vi "画箭头 - right.vi"(0 "Image 2":T1(plugin-control)=refnum, 5 "距离":dbl, 7 "Rectangle":T3={"Left"=793, "Top"=1130, "Right"=0, "Bottom"=0, "Rotation"=45.0} {"Rotation" format="%.2f"; "Left" scale=0.0..1024.0; "Right" scale=0.0..1024.0}, 9 "abgek":dbl, 11 "error in (no error)":errorcluster caption="错误输入（无错误）", 12 "long":sgl=300.0, 13 "Color 2":u32(colorbox)=16711680) -> (4 "Image out":T1(plugin-control), 15 "error out":errorcluster)   [LabVIEW 2017]
uses:
  <vilib>/Analysis/coordinate.llb/2D Cartesian Coordinate Shift (Array).vi
  <vilib>/Analysis/coordinate.llb/2D Cartesian Coordinate Rotation (Array).vi
  <vilib>/Analysis/NI_AALPro.lvlib
panel:
  in  "Width":u32=23
  out "添加的数组":T2[](array[typedef]) {"Y" format="%.2f"; "X" format="%.2f"}
  in  "Color":u32(colorbox)=16711680
  out "MiddleEndPoint":T2={"X"=892.0, "Y"=1299.75} {"Y" format="%.2f"; "X" format="%.2f"}
  out "MiddleStartPoint":T2={"X"=892.0, "Y"=1159.25} {"Y" format="%.2f"; "X" format="%.2f"}
  out "EndPoint":T2={"X"=892.0, "Y"=1370.0} {"Y" format="%.2f"; "X" format="%.2f"}
  out "StartPoint":T2={"X"=892.0, "Y"=1089.0} {"Y" format="%.2f"; "X" format="%.2f"}
  in  "sss":i32=30
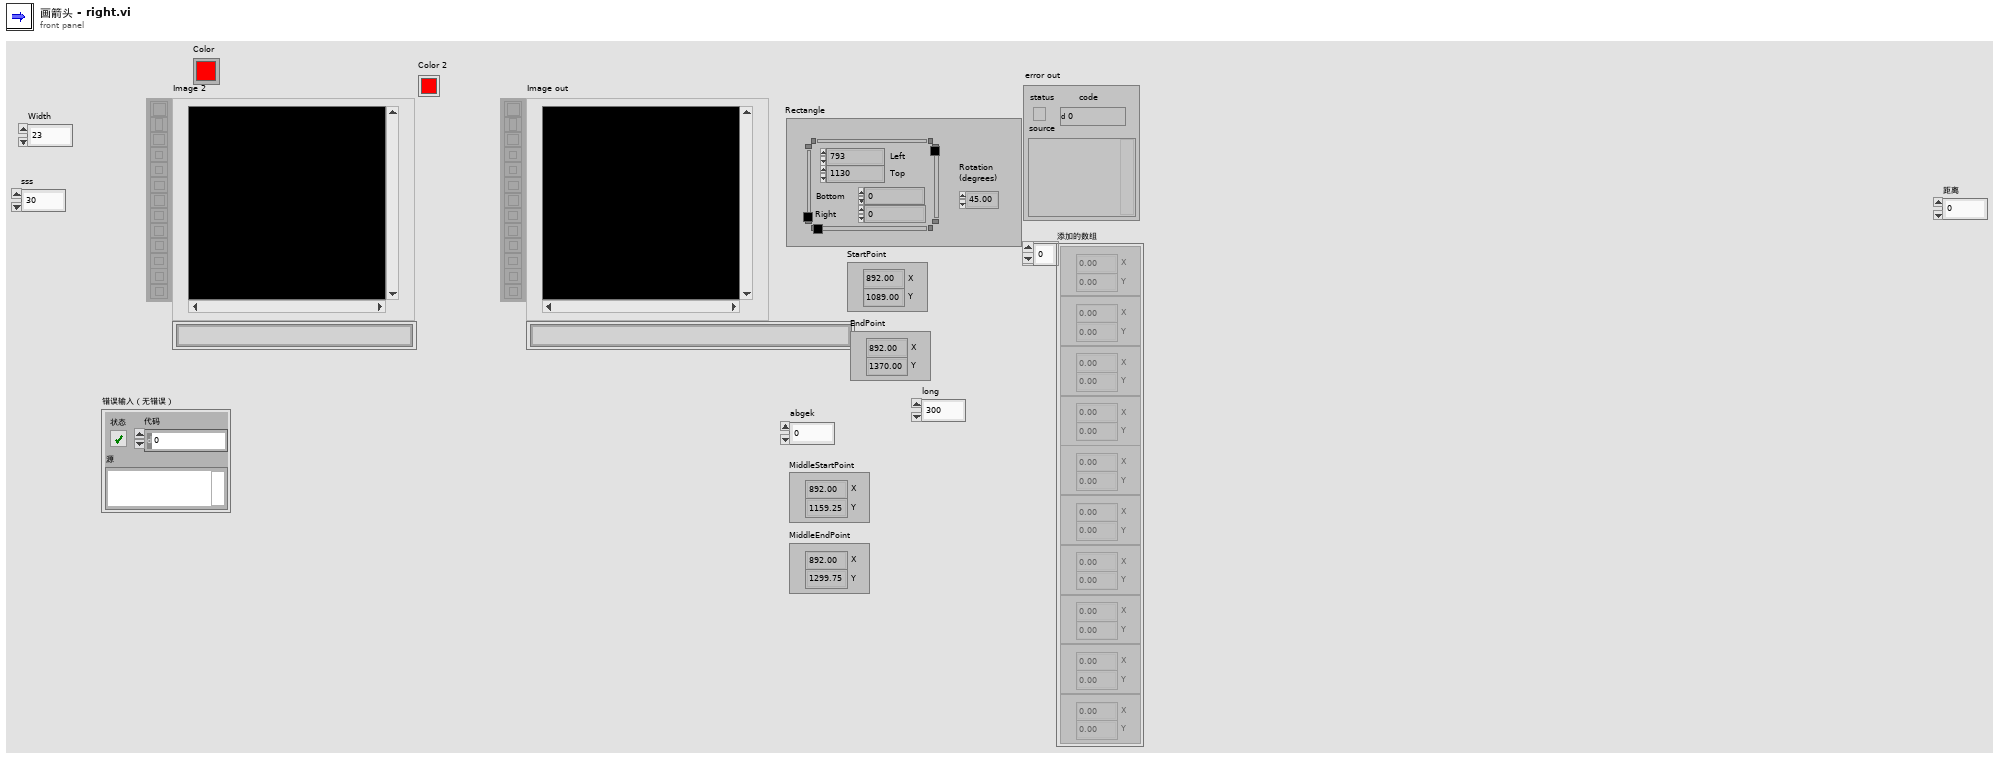
[diagram p1: front panel]
types:
  T1 = typedef "IMAQ Image.ctl" = refnum<image>
  T2 = typedef "IMAQ Point" = cluster{"X":sgl, "Y":sgl}
  T3 = typedef "IMAQ Rectangle" = cluster{"Left":i32, "Top":i32, "Right":i32, "Bottom":i32, "Rotation":dbl}
  T4 = cluster{"Desired Font (Application)":enum16{"User-specified Font", "Application Font", "System Font", "Dialog Font"}, "[User-specified Font]":cluster{"Font Name":string, "Size":i16, "Strikeout?":bool, "Italic?":bool, "Underline?":bool, "Outline?":bool, "Shadow?":bool, "Bold?":bool, "Rotation Angle":dbl}, "Horizontal Alignment":i16, "Vertical Alignment":i16}
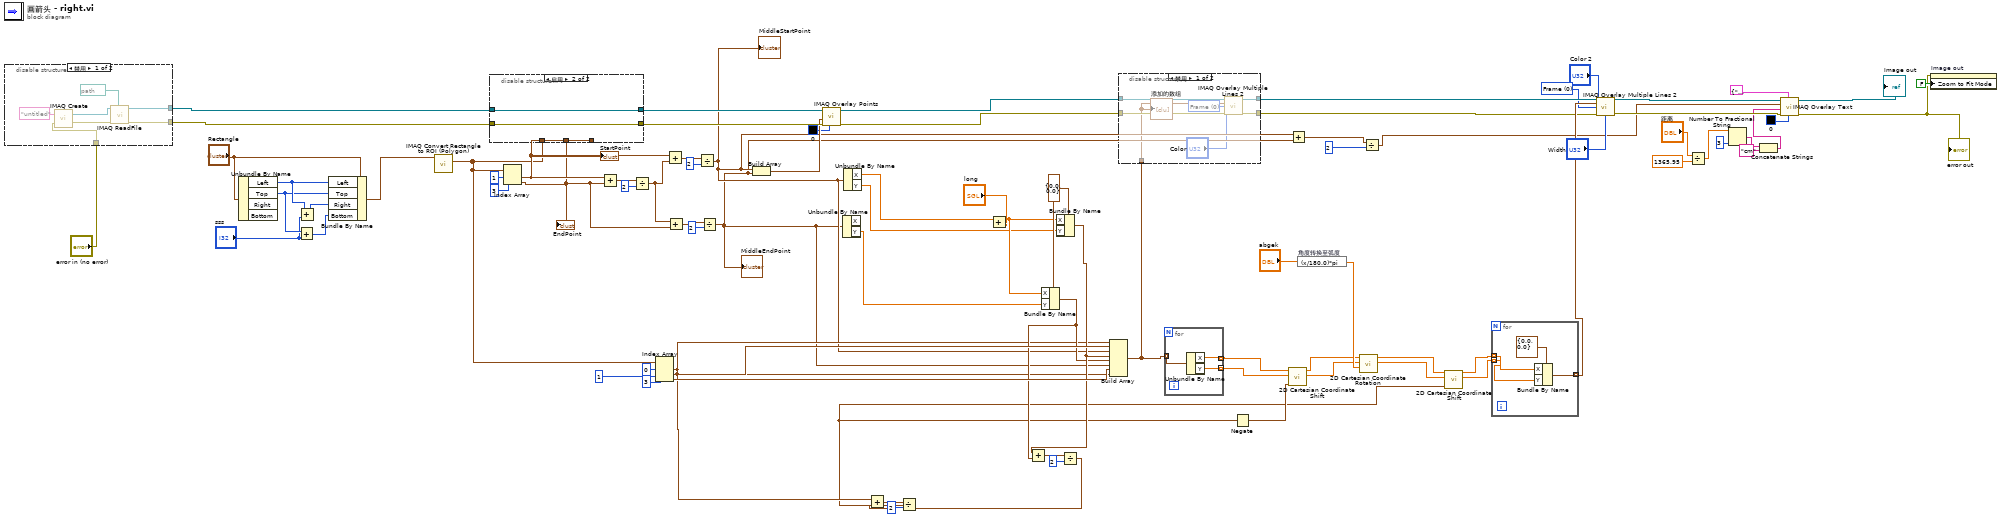
[diagram p0: block diagram]
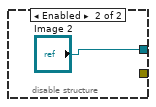
[diagram p2: hidden frame]
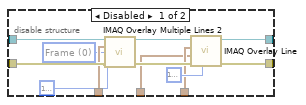
[diagram p4: hidden frame]
diagram:
  w34 = u32 0 items=["Frame", "Fill"] ("Drawing Mode (Frame)")
  w55 = T2 {"X"=0.0, "Y"=0.0} ("元素")
  n1 = disable-structure shown="禁用" {
    disable-tunnel: [w88 "Image 2"] -> w21
    disable-tunnel: [w87 _] -> w20
    disable-tunnel: "error in (no error)" -> [w86 _]
    frame Disabled {
      n2 = call "IMAQ Create"("Image Name"="untitled", "error in (no error)"=w86) -> ("New Image"=w90:T1, "error out"=w91:errorcluster)  [unwired: 3 in]
      n3 = call "IMAQ ReadFile"("File Path"=path "C:/Users/Lenovo/Desktop/PowerLine Inspect System/微信图片_20181113103336.bmp", "error in (no error)"=w91, "Image"=w90) -> ("error out"=w87:errorcluster, "Image Out"=w88:T1)  [unwired: 4 in, 3 out]
    }
    frame Enabled {
    }
  }
  n4 = Unbundle By Name("Rectangle") -> ("Left"=w83:i32, "Top"=w81:i32)  [unwired: 2 out]
  n5 = Add(x=w81, y="sss") -> (x+y=w79:i32)
  n6 = Add(x=w83, y="sss") -> (x+y=w82:i32)
  n7 = Bundle By Name(cluster="Rectangle", "Left"=w83, "Top"=w81, "Right"=w82, "Bottom"=w79) -> (w84:T3)
  n8 = call "IMAQ Convert Rectangle to ROI (Polygon)"("Rectangle"=w84) -> ("Rectangle Points"=w58:T2[])  [unwired: 7 in, 2 out]
  n9 = Index Array(array=w58, index #1=1 ("索引"), index #2=3 ("索引")) -> (element #1=w71:T2, element #2=w67:T2)
  "StartPoint" <- w71
  "EndPoint" <- w67
  n10 = disable-structure shown="启用" {
    disable-tunnel: w21 -> [w104 w107]
    disable-tunnel: w20 -> [w103 w106]
    disable-tunnel: [w102 w107] -> w78
    disable-tunnel: w71 -> [w99 _]
    disable-tunnel: w67 -> [w98 _]
    disable-tunnel: [w97 w106] -> w65
    disable-tunnel: w58 -> [w96 _]
    frame Disabled {
      w95 = u32 0 items=["Frame", "Fill"] ("Drawing Mode (Frame)")
      n11 = call "IMAQ Overlay Multiple Lines 2"("Image"=w104, "Line End Points"=w96, "Drawing Mode (Frame)"=w95, "Color"=u32 16777238, "error in (no error)"=w103) -> ("Image Out"=w105:T1, "error out"=w101:errorcluster)  [unwired: 9 in]
      n12 = call "IMAQ Overlay Line"("Color"=u32 16777238, "error in (no error)"=w101, "End Point"=w98, "Start Point"=w99, "Image"=w105) -> ("error out"=w97:errorcluster, "Image Out"=w102:T1)  [unwired: 5 in]
    }
    frame Enabled {
    }
  }
  n13 = Add(x=w71, y=w67) -> (x+y=w75:T2)
  n14 = Divide(x=w75, y=2) -> (x/y=w68:T2)
  n15 = Index Array(array=w58, index #1=0 ("索引"), index #2=1 ("索引"), index #3=3 ("索引")) -> (element #1=w26:T2, element #2=w57:T2, element #3=w49:T2)
  n16 = Add(x=w71, y=w68) -> (x+y=w72:T2)
  n17 = Add(x=w68, y=w67) -> (x+y=w70:T2)
  n18 = Divide(x=w72, y=2) -> (x/y=w11:T2)
  "MiddleStartPoint" <- w11
  n19 = Divide(x=w70, y=2) -> (x/y=w10:T2)
  "MiddleEndPoint" <- w10
  n20 = Build Array(w11, w10) -> (w64:T2[])
  n21 = call "IMAQ Overlay Points"("Color"=u32 0, "error in (no error)"=w65, "Array of Points"=w64, "Image"=w78) -> ("error out"=w61:errorcluster, "Image Out"=w66:T1)  [unwired: 6 in]
  n22 = Unbundle By Name(w10) -> ("Y"=w51:sgl)  [unwired: 1 out]
  n23 = Unbundle By Name(w11) -> ("X"=w56:sgl, "Y"=w52:sgl)
  n24 = Add(x=w56, y="long") -> (x+y=w54:sgl)
  n25 = Bundle By Name(cluster=w55, "X"=w54, "Y"=w51) -> (w28:T2)
  n26 = Bundle By Name(cluster=w55, "X"=w54, "Y"=w52) -> (w29:T2)
  n27 = Add(x=w29, y=w28) -> (x+y=w30:T2)
  n28 = Divide(x=w30, y=2) -> (x/y=w27:T2)
  n29 = Add(x=w26, y=w27) -> (x+y=w33:T2)
  n30 = Divide(x=w33, y=2) -> (x/y=w25:T2)
  n31 = Build Array(w26, w57, w11, w29, w28, w10, w49, w26) -> (w48:T2[])
  n32 = disable-structure shown="禁用" {
    disable-tunnel: w66 -> [w114 w116]
    disable-tunnel: [w113 w116] -> w62
    disable-tunnel: w61 -> [w112 w115]
    disable-tunnel: w48 -> [w111 _]
    disable-tunnel: [w110 w115] -> w44
    frame Disabled {
      w108 = u32 0 items=["Frame", "Fill"] ("Drawing Mode (Frame)")
      n33 = call "IMAQ Overlay Multiple Lines 2"("Image"=w114, "Line End Points"=w111, "Drawing Mode (Frame)"=w108, "Color"="Color", "error in (no error)"=w112) -> ("Image Out"=w113:T1, "error out"=w110:errorcluster)  [unwired: 9 in]
      "添加的数组" <- w111
    }
    frame Enabled {
    }
  }
  n34 = for {
    tunnel: w48 -> [w119] mode=indexing
    tunnel: [w118] -> w43 mode=indexing
    tunnel: [w117] -> w42 mode=indexing
    n35 = Unbundle By Name(w119) -> ("X"=w118:sgl, "Y"=w117:sgl)
  }
  n36 = Negate(x=w25) -> (-x=w41:T2)
  n37 = call-poly <vilib>:"2D Cartesian Coordinate Shift.vi"("shift"=w41, "Y"=w42, "X"=w43) -> ("Y Out"=w39:dbl[], "X Out"=w40:dbl[])  [unwired: 6 in, 1 out]
  n38 = Add(x=w11, y=w10) -> (x+y=w9:T2)
  n39 = expression code="(x/180.0)*pi" "角度转换至弧度"("abgek") -> (w46:dbl)
  n40 = call-poly <vilib>:"2D Cartesian Coordinate Rotation.vi"("theta"=w46, "Y"=w39, "X"=w40) -> ("Y Out"=w36:dbl[], "X Out"=w38:dbl[])  [unwired: 6 in, 1 out]
  n41 = Divide(x=w9, y=2) -> (x/y=w7:T2)
  n42 = call-poly <vilib>:"2D Cartesian Coordinate Shift.vi"("shift"=w25, "Y"=w36, "X"=w38) -> ("Y Out"=w35:dbl[], "X Out"=w37:dbl[])  [unwired: 6 in, 1 out]
  n43 = for {
    tunnel: w37 -> [w122] mode=indexing
    tunnel: w35 -> [w121] mode=indexing
    tunnel: [w120] -> w45 mode=indexing
    n44 = Bundle By Name(cluster=T2 {"X"=0.0, "Y"=0.0} ("元素"), "X"=w122, "Y"=w121) -> (w120:T2)
  }
  n45 = call "IMAQ Overlay Multiple Lines 2"("Image"=w62, "Line End Points"=w45, "Drawing Mode (Frame)"=w34, "Color"="Color 2", "error in (no error)"=w44, "Width"="Width") -> ("Image Out"=w15:T1, "error out"=w12:errorcluster)  [unwired: 8 in]
  n46 = Divide(x="距离", y=1365.95) -> (x/y=w4:dbl)
  n47 = Number To Fractional String(number=w4, precision (6)=i16 3 ("精度(6)")) -> (F-format string=w3:string)  [unwired: 2 in]
  n48 = Concatenate Strings(w3, "cm" ("字符串")) -> (w1:string)
  n49 = call "IMAQ Overlay Text"("Text Color (black)"=u32 0, "Font, Size & Style"=T4 {"Desired Font (Application)"=enum."User-specified Font", "[User-specified Font]"={"Font Name"="", "Size"=15, "Strikeout?"=FALSE, "Italic?"=FALSE, "Underline?"=FALSE, "Outline?"=FALSE, "Shadow?"=FALSE, "Bold?"=TRUE, "Rotation Angle"=0.0}, "Horizontal Alignment"=1, "Vertical Alignment"=0}, "error in (no error)"=w12, "String"=w1, "Origin"=w7, "Image"=w15) -> ("error out"=w13:errorcluster, "Image Out"=→"Image out":T1)  [unwired: 4 in]
  "error out" <- w13
  n50 = property on="Image out" class="ImageControl"(error in=w13, "Zoom to Fit Mode"=FALSE) -> ()  [unwired: 1 in, 2 out]
